vi "HFRR ADV v044.vi"() -> ()   [LabVIEW 2025] (continued)
            "LVDT MIN" <- w2060
            "LVDT MAX" <- w2059
            "LVDT Peak" <- w2058
            "pizo raw" <- w2057
            "cof" <- w2055
            "Frictioin Force Raw" <- w2056
          }
        }
      }
      frame Error {
      }
    }
    n1795 = local read "Quit"() -> (w1974:bool)
  }
  n1796 = disable-structure shown="Disabled" {
    disable-tunnel: errorcluster {"status"=TRUE, "code"=0, "source"="Init"} ("error IO") -> [w2119 _]
    disable-tunnel: [w2117 _] -> w50
    frame Disabled {
      n1797 = while {
        shift-right: [w2135] -> w2121
        shift-left: _ -> [w2126]
        shift-right: [w2134] -> w2120
        shift-left: w2119 -> [w2128]
        tunnel: [w2123] -> w2117
        tunnel: [w2133] -> _
        i -> [w2133]
        stop <- w2123 stop-if-true
        n1798 = local read "Port 1a"() -> (w2129:bool)
        n1799 = local read "Port 3"() -> (w2130:bool)
        n1800 = local read "Com Port 1"() -> (w2127:refnum<visa-resource-name>)
        n1801 = Or(x=w2130, y=w2129) -> (x .or. y?=w2132:bool)
        n1802 = Unbundle(w2128) -> ("status"=→"Port 3":bool)  [unwired: 2 out]
        n1803 = Not Equal?(x=w2127, y=w2126) -> (x != y?=w2124:bool)
        n1804 = case shown="True" w2132 {
          frame False {
            w2138 = TRUE ("Visible")
            n1805 = property on="Port 1a" class="Bool (strict)"("Visible"=w2138) -> ()  [unwired: 2 in, 2 out]
            n1806 = property on="Port 3" class="Bool (strict)"("Visible"=w2138) -> ()  [unwired: 2 in, 2 out]
          }
          frame True {
            w2139 = TRUE ("Visible")
            n1807 = property on="Port 1a" class="Bool (strict)"("Visible"=w2139) -> ()  [unwired: 2 in, 2 out]
            n1808 = property on="Port 3" class="Bool (strict)"("Visible"=w2139) -> ()  [unwired: 2 in, 2 out]
          }
        }
        n1809 = Wait (ms)(milliseconds to wait=u32 40) -> ()  [unwired: 1 out]
        n1810 = case shown="True" w2124 {
          tunnel: [w2136 errorcluster {"status"=TRUE, "code"=0, "source"="Init"} ("error out")] -> w2125
          tunnel: w2128 -> [w2136 _]
          frame False {
          }
          frame True {
          }
        }
        n1811 = case shown="Error" w2125 {
          selector: w2125 -> [w2146 w2164]
          tunnel: [w2149 w2168] -> w2135
          tunnel: [w2148 w2162] -> w2134
          tunnel: w2126 -> [w2147 w2166]
          frame No Error {
            n1812 = property class="Instr"(reference=w2147, error in=w2146) -> (reference out=w2144:refnum<visa-resource-name>, error out=w2145:errorcluster, "Serial Settings:Number of Bytes at Serial Port"=w2141:u32)
            n1813 = Greater?(x=w2141, y=u32 5) -> (0:w2140:bool)
            n1814 = Not(x=w2140) -> (.not. x?=→"Port 1a":bool)
            n1815 = while {
              tunnel: [w2157] -> w2148
              tunnel: [w2156] -> w2149
              tunnel: w2145 -> [w2155]
              tunnel: w2144 -> [w2154]
              stop <- TRUE stop-if-true
              n1816 = property class="Instr" props=["Serial Settings:Number of Bytes at Serial Port"](reference=w2154, error in=w2155) -> (reference out=w2159:refnum<visa-resource-name>, error out=w2158:errorcluster)  [unwired: 1 out]
              n1817 = VISA Read(VISA resource name=w2159, byte count=u32 50, error in (no error)=w2158) -> (VISA resource name out=w2156:refnum<visa-resource-name>, read buffer=w2151:string, error out=w2157:errorcluster)  [unwired: 1 out]
              n1818 = Wait (ms)(milliseconds to wait=u32 5) -> ()  [unwired: 1 out]
            }
          }
          frame Error {
            w2174 = u16 0 items=["None", "XON/XOFF", "RTS/CTS", "XON/XOFF & RTS/CTS", "DTR/DSR", "XON/XOFF & DTR/DSR"] ("flow control (0:none)  2")
            w2172 = u16 10 items=["1.0"=10, "1.5"=15, "2.0"=20] ("stop bits 2")
            w2170 = u16 0 items=["None", "Odd", "Even", "Mark", "Space"] ("parity 2")
            w2171 = u32 10000  # timeout (10sec)
            n1819 = VISA Close(VISA resource name=w2166, error in (no error)=w2164) -> (error out=w2167:errorcluster)
            n1820 = local write "Port 1a"(FALSE ("Port 1a")) -> ()
            n1821 = local read "Com Port 1"() -> (w2161:refnum<visa-resource-name>)
            n1822 = call <vilib>:"Clear Errors.vi"("error in (no error)"=w2167) -> ("error out"=w2165:errorcluster)  [unwired: 5 in, 1 out]
            n1823 = call-poly "VISA Configure Serial Port"("VISA resource name"=w2161, "timeout (10sec)"=w2171, "baud rate (9600)"=u32 250000 ("baud rate  2"), "data bits (8)"=u16 8 ("data bits  2"), "parity (0:none)"=w2170, "error in (no error)"=w2165, "stop bits (10: 1 bit)"=w2172, "flow control (0:none)"=w2174) -> ("VISA resource name out"=w2175:refnum<visa-resource-name>, "error out"=w2176:errorcluster)  [unwired: 6 in]
            n1824 = flat-sequence {
              tunnel: w2175 -> [w2178]
              tunnel: w2176 -> [w2177]
              tunnel: [w2178] -> w2168
              tunnel: [w2177] -> w2162
              frame #0 {
                n1825 = Wait (ms)(milliseconds to wait=u32 50) -> ()  [unwired: 1 out]
              }
            }
            "Residual Uno" <- ""
          }
        }
        n1826 = local read "Quit"() -> (w2123:bool)
        "Error Uno" <- w2128
      }
      n1827 = VISA Close(VISA resource name=w2121, error in (no error)=w2120) -> (error out=w2118:errorcluster)
      n1828 = call <vilib>:"Clear Errors.vi"("error in (no error)"=w2118) -> ()  [unwired: 5 in, 2 out]
    }
    frame Enabled {
    }
  }
  n1829 = while {
    stop <- w2189 stop-if-true
    # "V0OLTAGE TO STROKE (peice vise calibration)"
    n1830 = local read "LVDT MIN"() -> (w2181:dbl)
    n1831 = local read "LVDT Peak"() -> (w2180:dbl)
    n1832 = Wait (ms)(milliseconds to wait=u32 10) -> ()  [unwired: 1 out]
    n1833 = formula code="// Dynamic Parameterized Linear Interpolation Node\n// Inputs: vpp_val, voltages (Array), distances (Array)\n// Outputs: stroke\n\nint i = 0;\nint segments = 11; // 12 points make 11 interpolation segments\n\n// 1. Lower Boundary Clamp\nif (vpp_val <= voltages[0]) {\n    stroke = distances[0];\n}\n// 2. Upper Boundary Clamp\nelse if (vpp_val >= voltages[segments]) {\n    stroke = distances[segments];\n}\n// 3. Dynamic Segment Search Loop\nelse {\n    stroke = distances[0]; // Fallback baseline\n    for (i = 0; i < segments; i++) {\n        if (vpp_val >= voltages[i] && vpp_val <= voltages[i+1]) {\n            // Standard linear interpolation formula using array lookups\n            stroke = distances[i] + (vpp_val - voltages[i]) * (distances[i+1] - distances[i]) / (voltages[i+1] - voltages[i]);\n            break; // Segment found, safely exit the loop\n        }\n    }\n}"("vpp_val"=w2180, "voltages"="calibration values", "distances"="STROKE") -> ("stroke"=→"LVDT STROKE":dbl)
    n1834 = local read "Calibration Tare Value"() -> (w2185:dbl)
    n1835 = local read "Calibration Tare"() -> (w2183:bool)
    n1836 = Subtract(x=w2181, y=w2185) -> (x-y=→"LVDT STROKE  Calibration":dbl)
    n1837 = case shown="True" w2183 {
      selector: w2183 -> [_ w2191]
      tunnel: w2181 -> [_ w2192]
      frame False {
      }
      frame True {
        n1838 = Not(x=w2191) -> (.not. x?=w2190:bool)
        n1839 = local write "Calibration Tare"(w2190) -> ()
        "Calibration Tare Value" <- w2192
      }
    }
    n1840 = local read "Quit"() -> (w2189:bool)
  }
  n1841 = while {
    stop <- w2215 stop-if-true
    n1842 = local read "Due read"() -> (w2213:string)
    n1843 = call <vilib>:"High Resolution Polling Wait.vi"("seconds to wait"=0.02) -> ()  [unwired: 10 in, 1 out]
    n1844 = local read "Frictioin Force Raw"() -> (w2195:dbl)
    n1845 = Spreadsheet String To Array(delimiter (Tab)=";", format string="", spreadsheet string=w2213, array type (2D Dbl)=string[] []) -> (array=w2210:string[])
    n1846 = Fract/Exp String To Number(string=w2210) -> (number=w2209:dbl[])  [unwired: 3 in, 1 out]
    n1847 = call <vilib>:"Median Filter PtByPt.vi"("rank"=2, "x"=w2195) -> ("Filtered x"=→"Friction":dbl)  [unwired: 2 in, 1 out]
    n1848 = Index Array(array=w2209) -> (element #1=→"Sample Temperature 2":dbl, element #2=→"Target Sample Temperature":dbl, element #3=→"Current Duty Cycle":dbl, element #4=→"Ambient Temperature":dbl, element #5=→"Dac Status":dbl, element #6=→"Vpp":dbl, element #7=→"Active Error Code":dbl, element #8=→"Kp":dbl, element #9=→"Ki":dbl, element #10=→"Kd":dbl, element #11=→"SampleRaw":dbl, element #12=→"AmbRaw":dbl)  [unwired: 12 in]
    n1849 = local read "Quit"() -> (w2215:bool)
  }
  n1850 = while {
    shift-right: [w2229] -> w46
    shift-left: _ -> [w2221]
    shift-right: [w2216] -> w45
    shift-left: errorcluster {"status"=FALSE, "code"=0, "source"="Init"} ("error out") -> [w2223]
    tunnel: [w2218] -> w49
    tunnel: [w2228] -> _
    i -> [w2228]
    stop <- w2218 stop-if-true
    n1851 = local read "Com Port 2"() -> (w2222:refnum<visa-resource-name>)
    n1852 = local read "Port 2a"() -> (w2224:bool)
    n1853 = Unbundle(w2223) -> ("status"=→"Port 4":bool)  [unwired: 2 out]
    n1854 = call <vilib>:"High Resolution Polling Wait.vi"("seconds to wait"=0.02) -> ()  [unwired: 10 in, 1 out]
    n1855 = local read "Port 4"() -> (w2225:bool)
    n1856 = Not Equal?(x=w2222, y=w2221) -> (x != y?=w2220:bool)
    n1857 = Or(x=w2225, y=w2224) -> (x .or. y?=w2227:bool)
    n1858 = case shown="False" w2227 {
      frame False {
        w2232 = TRUE ("Visible")
        n1859 = property on="Port 2a" class="Bool (strict)"("Visible"=w2232) -> ()  [unwired: 2 in, 2 out]
        n1860 = property on="Port 4" class="Bool (strict)"("Visible"=w2232) -> ()  [unwired: 2 in, 2 out]
      }
      frame True {
        w2233 = TRUE ("Visible")
        n1861 = property on="Port 2a" class="Bool (strict)"("Visible"=w2233) -> ()  [unwired: 2 in, 2 out]
        n1862 = property on="Port 4" class="Bool (strict)"("Visible"=w2233) -> ()  [unwired: 2 in, 2 out]
      }
    }
    n1863 = case shown="True" w2220 {
      tunnel: [w2230 errorcluster {"status"=TRUE, "code"=0, "source"="Init"} ("error out")] -> w2219
      tunnel: w2223 -> [w2230 _]
      frame False {
      }
      frame True {
      }
    }
    n1864 = case shown="No Error" w2219 {
      selector: w2219 -> [w2246 w2277]
      tunnel: [w2239 w2282] -> w2229
      tunnel: [w2247 w2275] -> w2216
      tunnel: w2221 -> [w2248 w2280]
      frame No Error {
        n1865 = property class="Instr" props=["Serial Settings:Number of Bytes at Serial Port"](reference=w2248, error in=w2246) -> (reference out=w2240:refnum<visa-resource-name>, error out=w2245:errorcluster)  [unwired: 1 out]
        n1866 = while {
          tunnel: [w2256] -> w2241
          tunnel: [w2255] -> w2242
          tunnel: w2245 -> [w2254]
          tunnel: w2240 -> [w2253]
          tunnel: [w2252] -> _
          i -> [w2252]
          stop <- TRUE stop-if-true
          n1867 = property class="Instr" props=["Serial Settings:Number of Bytes at Serial Port"](reference=w2253, error in=w2254) -> (reference out=w2258:refnum<visa-resource-name>, error out=w2257:errorcluster)  [unwired: 1 out]
          n1868 = VISA Read(VISA resource name=w2258, byte count=u32 1000, error in (no error)=w2257) -> (VISA resource name out=w2255:refnum<visa-resource-name>, read buffer=→"Due read":string, error out=w2256:errorcluster)  [unwired: 1 out]
        }
        n1869 = local read "Due Write"() -> (w2238:string)
        n1870 = call <vilib>:"Trim Whitespace.vi"("string"=w2238) -> ("trimmed string"=w2237:string)  [unwired: 1 in]
        n1871 = Not Equal?(x=w2237, y="") -> (x != y?=w2243:bool)
        n1872 = VISA Flush I/O Buffer(VISA resource name=w2242) -> (VISA resource name out=w2235:refnum<visa-resource-name>, error out=→"error out 10":errorcluster)  [unwired: 2 in]
        n1873 = case shown="True" w2243 {
          tunnel: w2235 -> [w2260 w2265]
          tunnel: [w2260 w2269] -> w2239
          tunnel: w2241 -> [w2259 w2264]
          tunnel: [w2259 w2267] -> w2247
          tunnel: w2237 -> [_ w2263]
          tunnel: [_ w2266] -> _
          frame False {
            # "DATA  WRITE LOOP"
          }
          frame True {
            n1874 = Concatenate Strings(w2263, "\r\n") -> (w2262:string)
            n1875 = VISA Write(VISA resource name=w2265, write buffer=w2262, error in (no error)=w2264) -> (VISA resource name out=w2269:refnum<visa-resource-name>, return count=w2266:u32, error out=w2268:errorcluster)
            n1876 = flat-sequence {
              tunnel: w2268 -> [w2271]
              tunnel: [w2271] -> w2267
              frame #0 {
                n1877 = local write "Due Write"("" ("Command")) -> ()
                n1878 = Wait (ms)(milliseconds to wait=u32 5) -> ()  [unwired: 1 out]
              }
            }
          }
        }
        "Port 2a" <- TRUE ("Port 2a")
      }
      frame Error {
        w2288 = u16 0 items=["None", "XON/XOFF", "RTS/CTS", "XON/XOFF & RTS/CTS", "DTR/DSR", "XON/XOFF & DTR/DSR"] ("flow control (0:none)  2")
        w2286 = u16 10 items=["1.0"=10, "1.5"=15, "2.0"=20] ("stop bits 2")
        w2284 = u16 0 items=["None", "Odd", "Even", "Mark", "Space"] ("parity 2")
        w2285 = u32 10000  # timeout (10sec)
        n1879 = VISA Clear(VISA resource name=w2280, error in (no error)=w2277) -> (VISA resource name out=w2279:refnum<visa-resource-name>, error out=w2278:errorcluster)
        n1880 = VISA Close(VISA resource name=w2279, error in (no error)=w2278) -> (error out=w2281:errorcluster)
        n1881 = call <vilib>:"Clear Errors.vi"("error in (no error)"=w2281) -> ()  [unwired: 5 in, 2 out]
        n1882 = local write "Port 2a"(FALSE ("Port 2a")) -> ()
        n1883 = local read "Com Port 2"() -> (w2274:refnum<visa-resource-name>)
        "visa due" <- w2274
        n1884 = call-poly "VISA Configure Serial Port"("VISA resource name"=w2274, "timeout (10sec)"=w2285, "baud rate (9600)"=u32 250000 ("baud rate  2"), "data bits (8)"=u16 8 ("data bits  2"), "parity (0:none)"=w2284, "stop bits (10: 1 bit)"=w2286, "flow control (0:none)"=w2288) -> ("VISA resource name out"=w2289:refnum<visa-resource-name>, "error out"=w2290:errorcluster)  [unwired: 7 in]
        n1885 = flat-sequence {
          tunnel: w2289 -> [w2292]
          tunnel: w2290 -> [w2291]
          tunnel: [w2292] -> w2282
          tunnel: [w2291] -> w2275
          frame #0 {
            n1886 = Wait (ms)(milliseconds to wait=u32 50) -> ()  [unwired: 1 out]
          }
        }
        "Residual Due" <- ""
      }
    }
    "error out 9" <- w2216
    n1887 = local read "Quit"() -> (w2218:bool)
    "Error Due" <- w2223
  }
  n1888 = local write "FRICVALZ"(0.0 ("FRICVALZ")) -> ()
  n1889 = property on="RUN" class="Bool (strict)"("Visible"=TRUE) -> ()  [unwired: 2 in, 2 out]
  n1890 = while {
    tunnel: [w2307] -> _
    tunnel: [w2294] -> w59
    i -> [w2307]
    stop <- w2294 stop-if-true
    n1891 = local read "conststatus"() -> (w2298:dbl)
    n1892 = local read "Main Tab"() -> (w2296:T4)
    n1893 = local read "EDIT"() -> (w2313:bool)
    n1894 = local read "Rate"() -> (w2312:dbl)
    n1895 = case shown="True" w2313 {
      tunnel: [FALSE TRUE] -> _
      frame False {
      }
      frame True {
      }
    }
    n1896 = Equal?(x=w2296, y=T28."About" ("Main Tab")) -> (x = y?=w2305:bool)
    n1897 = Equal?(x=w2298, y=0.0) -> (x = y?=w2299:bool)
    n1898 = Divide(x=1.0, y=w2312) -> (x/y=w2308:dbl)
    "Time 2" <- w2308
    n1899 = case shown="True" w2299 {
      frame False {
      }
      frame True {
        # "C:\\WinDucom\\calibrate WO 2391.dcf"
        n1900 = local write "Lan flag"(22) -> ()
        n1901 = local write "conststatus"(10.0 ("rpm value : 2")) -> ()
        n1902 = String To Path(string="C:\\LAB-IQ\\calibrate WO 2465.dcf") -> (path=w2319:path)
        n1903 = Open/Create/Replace File "Open File"(file path (use dialog)=w2319) -> (refnum out=w2317:refnum<file>)  [unwired: 5 in, 2 out]
        n1904 = for {
          N: 23 -> [_]
          tunnel: w2317 -> [w2328]
          i -> [w2322]
          (unwired) TRUE ("line mode (F)")
          n1905 = Read from Text File "Read File"(file (use dialog)=w2328) -> (text=w2327:string)  [unwired: 3 in, 3 out]
          n1906 = Match Pattern(string=w2327, regular expression="]") -> (after substring=w2325:string)  [unwired: 1 in, 3 out]
          n1907 = String Subset(string=w2327, offset (0)=5, length (rest)=10 ("length (rest)")) -> (substring=w2320:string)
          n1908 = Fract/Exp String To Number(string=w2320) -> (number=w2321:dbl)  [unwired: 3 in, 1 out]
          n1909 = Match Pattern(string=w2325, regular expression="-") -> (before substring=w2323:string)  [unwired: 1 in, 3 out]
          n1910 = case shown="10" w2322 {
            tunnel: w2321 -> [_ _ _ _ _ _ _ _ _ _ w2335 _ _ _ _ _ _ _ _ _ _ _ _ _]
            tunnel: w2323 -> [_ _ _ _ w2331 w2332 w2333 _ _ _ _ _ _ _ _ _ _ _ _ _ w2336 w2337 w2338 _]
            frame 0 {
            }
            frame 1 {
            }
            frame 2 {
            }
            frame 3 {
            }
            frame 4 {
              n1911 = local write "Com Port 1"(w2331) -> ()
            }
            frame 5 {
              n1912 = local write "Com Port 2"(w2332) -> ()
              n1913 = local write "visa due"(w2332) -> ()
            }
            frame 6 {
              n1914 = String To Path(string=w2333) -> (path=w2334:path)
              n1915 = local write "File Path"(w2334) -> ()
              "String" <- w2333
            }
            frame 7 {
            }
            frame 8 {
            }
            frame 9 {
            }
            frame 10 {
              n1916 = local write "Language Selection"(w2335) -> ()
            }
            frame 11 {
            }
            frame 12 {
            }
            frame 13 {
            }
            frame 14 {
            }
            frame 15 {
            }
            frame 16 {
            }
            frame 17 {
            }
            frame 18 {
            }
            frame 21 {
            }
            frame 22 {
              n1917 = local write "Com Port 3"(w2336) -> ()
            }
            frame 20 {
              n1918 = local write "Camera Port :"(w2337) -> ()
            }
            frame 19 {
              n1919 = local write "C3 :"(w2338) -> ()
            }
            frame 23, Default {
            }
          }
        }
      }
    }
    n1920 = Select(t=u32 2500 ("milliseconds to wait"), s=w2305, f=u32 500 ("milliseconds to wait")) -> (s? t:f=w2303:u32)
    n1921 = Multiply(x=w2308, y=w2303) -> (x*y=w2310:dbl)
    n1922 = call "Elapsed Time2"("Time Target (s)"=w2310, "Auto Reset"=TRUE) -> ("Time has Elapsed"=w2300:bool)  [unwired: 10 in, 7 out]
    n1923 = case shown="True" w2300 {
      frame False {
      }
      frame True {
        n1924 = stacked-sequence {
          frame #0 {
            # "DATA PROCESSING"
            # "115 mV/N"
            n1925 = local read "Sample Temperature 2"() -> (w2341:dbl)
            n1926 = local read "RH Numeric:"() -> (→"Humidity ( %RH )":dbl)
            n1927 = local read "FRICVALZ"() -> (w2358:dbl)
            n1928 = local read "Friction"() -> (w2344:dbl)
            n1929 = call <vilib>:"Mean PtByPt.vi"("x"=w2341, "sample length"=100) -> ("mean"=w2340:dbl)  [unwired: 2 in, 1 out]
            "TEMP 2" <- w2340
            "TEMP 3" <- w2340
            n1930 = Subtract(x=w2344, y=w2358) -> (x-y=w2353:dbl)
            "FF 2" <- w2353
            "FF 4" <- w2353
            n1931 = local read "Ambient Temperature"() -> (→"AIR TEMP":dbl)
            n1932 = local read "TEMP"() -> (w2357:dbl)
            n1933 = local write "FF 3"(w2353) -> ()
            n1934 = Compound Arithmetic op=OR("FRICVALZ 4", "FRICVALZ 3", "FRICVALZ 2") -> (w2349:bool)
            n1935 = case shown="True" w2349 {
              tunnel: w2344 -> [_ w2364]
              frame False {
              }
              frame True {
                w2363 = FALSE ("FRICVALZ")
                n1936 = local write "FRICVALZ 3"(w2363) -> ()
                n1937 = local write "FRICVALZ 2"(w2363) -> ()
                n1938 = local write "FRICVALZ 4"(w2363) -> ()
                "FRICVALZ" <- w2364
              }
            }
            n1939 = Not A Number/Path/Refnum?(number/path/refnum=w2357) -> (NaN/Path/Refnum?=w2356:bool)
            n1940 = Not A Number/Path/Refnum?(number/path/refnum=w2353) -> (NaN/Path/Refnum?=w2355:bool)
            n1941 = Divide(x=w2353, y=1.96) -> (x/y=w2350:dbl)
            n1942 = Compound Arithmetic op=OR(w2356, w2355) -> (w2354:bool)
            n1943 = Not A Number/Path/Refnum?(number/path/refnum=w2350) -> (NaN/Path/Refnum?=w2351:bool)
            n1944 = case shown="True" w2354 {
              frame False {
              }
              frame True {
                n1945 = local write "TEMP"(0.0 ("TEMP")) -> ()
                n1946 = local write "FF 2"(0.0 ("FF 2")) -> ()
                n1947 = local write "reinit"(TRUE ("reinit")) -> ()
              }
            }
            n1948 = local write "TEMP"(w2340) -> ()
            n1949 = Select(t=0.0, s=w2351, f=w2350) -> (s? t:f=w2343:dbl)
            "COF 2" <- w2343
            n1950 = local write "COF 3"(w2343) -> ()
          }
        }
      }
    }
    n1951 = Wait (ms)(milliseconds to wait=u32 50) -> ()  [unwired: 1 out]
    n1952 = local read "Quit"() -> (w2294:bool)
    "Rate" <- 2500.0 ("No of Samples")
  }
  n1953 = while {
    tunnel: [w2384] -> _
    tunnel: [w2367] -> w61
    tunnel: w6 -> [_]
    i -> [w2384]
    stop <- w2367 stop-if-true
    # "C:\\LAB-IQ-NXT\\Scar View.exe"
    n1954 = local read "OK Button 16"() -> (w2374:bool)
    n1955 = local read "Main Tab"() -> (w2368:T4)
    n1956 = local read "service 3"() -> (w2369:bool)
    n1957 = local read "OPEN 6"() -> (w2371:bool)
    n1958 = local read "EDIT 2"() -> (w2373:bool)
    n1959 = flat-sequence {
      frame #0 {
        n1960 = stacked-sequence {
          frame #0 {
            n1961 = local read "EDIT"() -> (w2862:bool)
            n1962 = case shown="False" w2862 {
              tunnel: [u8 2 ("Disabled") u8 0 ("Disabled")] -> _
              frame False {
                w2864 = FALSE
                n1963 = local write "Password"("") -> ()
                n1964 = local write "x = y?"(w2864) -> ()
                n1965 = property on="Password" class="Str"("Visible"=w2864) -> ()  [unwired: 2 in, 2 out]
              }
              frame True {
                n1966 = property on="Password" class="Str"("Visible"=TRUE) -> ()  [unwired: 2 in, 2 out]
              }
            }
            "dipl pwd" <- "@143$\n" ("dipl pwd")
          }
          frame #1 {
          }
          frame #2 {
          }
          frame #3 {
          }
          frame #4 {
            n1967 = String To Byte Array(string="Password") -> (unsigned byte array=w2875:u8[])
            n1968 = Search 1D Array(1D array=w2875, element=u8 10) -> (index of element=w2873:i32)  [unwired: 1 in]
            n1969 = Index Array(array=w2875, index=w2873) -> (element=w2874:u8)
            n1970 = Equal?(x=w2874, y=10) -> (x = y?=w2870:bool)
            n1971 = case shown="True" w2870 {
              frame False {
              }
              frame True {
                # "password"
                # "password"
                n1972 = local read "Password"() -> (w2887:string)
                n1973 = String To Byte Array(string=w2887) -> (unsigned byte array=w2890:u8[])
                n1974 = String To Byte Array(string="@143$\n") -> (unsigned byte array=w2877:u8[])
                n1975 = Array Size(array=w2890) -> (size(s)=w2886:i32)
                n1976 = Array Size(array=w2877) -> (size(s)=w2882:i32)
                n1977 = for {
                  N: w2886 -> [_]
                  tunnel: w2890 -> [w2903]
                  tunnel: [w2901] -> w2891 mode=indexing
                  tunnel: w2886 -> [w2898]
                  i -> [w2899]
                  n1978 = Decrement(x=w2898) -> (x-1=w2897:i32)
                  n1979 = Index Array(array=w2903, index=w2899) -> (element=w2902:u8)
                  n1980 = Equal?(x=w2899, y=w2897) -> (x = y?=w2896:bool)
                  n1981 = Number To Decimal String(number=w2902) -> (decimal integer string=w2900:string)  [unwired: 1 in]
                  n1982 = Select(t="", s=w2896, f="\r") -> (s? t:f=w2893:string)
                  n1983 = Concatenate Strings(w2900, w2893) -> (w2901:string)
                }
                n1984 = for {
                  N: w2882 -> [_]
                  tunnel: w2877 -> [w2914]
                  tunnel: [w2912] -> w2880 mode=indexing
                  tunnel: w2882 -> [w2909]
                  i -> [w2910]
                  n1985 = Decrement(x=w2909) -> (x-1=w2908:i32)
                  n1986 = Index Array(array=w2914, index=w2910) -> (element=w2913:u8)
                  n1987 = Equal?(x=w2910, y=w2908) -> (x = y?=w2907:bool)
                  n1988 = Number To Decimal String(number=w2913) -> (decimal integer string=w2911:string)  [unwired: 1 in]
                  n1989 = Select(t="", s=w2907, f="\r") -> (s? t:f=w2904:string)
                  n1990 = Concatenate Strings(w2911, w2904) -> (w2912:string)
                }
                n1991 = local read "file path"() -> (w2876:path)
                n1992 = call <vilib>:"Read Characters From File.vi"("file path (dialog if empty)"=w2876) -> ("character string"=w2889:string)  [unwired: 5 in, 3 out]
                "string" <- w2889
                n1993 = flat-sequence {
                  tunnel: [w2892] -> _
                  frame #0 {
                    w2892 = ""
                    n1994 = local write "Password"(w2892) -> ()
                  }
                }
                n1995 = Concatenate Strings(w2880) -> (w2881:string)
                n1996 = Concatenate Strings(w2889) -> (w2888:string)
                n1997 = Concatenate Strings(w2891) -> (w2884:string)
                n1998 = Equal?(x=w2884, y=w2888) -> (x = y?=w2879:bool)
                n1999 = Equal?(x=w2884, y=w2881) -> (x = y?=w2885:bool)
                n2000 = Or(x=w2879, y=w2885) -> (x .or. y?=→"x = y?":bool)
              }
            }
          }
        }
        n2001 = local read "x = y?"() -> (w2860:bool)
        n2002 = And(x="EDIT", y=w2860) -> (x .and. y?=w2858:bool)
        n2003 = case shown="True" w2858 {
          tunnel: [u8 2 ("Disabled") u8 0 ("Disabled")] -> w2857
          tunnel: [w3064 TRUE ("Visible")] -> w2856
          frame False {
            w3064 = FALSE ("Visible")
            n2004 = local write "EDIT 2"(w3064) -> ()
          }
          frame True {
          }
        }
        n2005 = case shown="True" "SAVE" {
          frame False {
          }
          frame True {
            n2006 = stacked-sequence {
              seq-local: [w2919 _ _] -> [_ w3060 _]
              frame #0 {
                w2915 = 0.0 ("number")
                w2916 = 0.0 ("number")
                (unwired) i16 5 ("precision (6)")
                # "[CH1]    - FF\n[CH2]   - TEMPERATURE\n[CH3]    - Humidity\n[CH4]    - AIR TEMP\n[CH5]\\- Visa Uno\n[CH6] \\- Visa Due\n[CH7]  \\- file path\n[CH8]   - Displacement Gain\n[CHA]   - Stroke Gain\n[CHB]   - Stroke PID Gain\n[CHC]   -Language Selection\n[CHD]   -Power +\n[CHE]   -Power_\n[CHF]   -Heater\n[CHG]   -Humidity Wet\n[CHH]   -Humidity Dry\n[CHI]   -Integral Time"
                n2007 = local read "Language Selection"() -> (w2962:enum16{"English", "Russian"})
                n2008 = Path To String(path="File Path") -> (string=w2978:string)
                n2009 = Number To Fractional String(number=w2915, width (-)=i16 10 ("precision (6)"), precision (6)=i16 5) -> (F-format string=w2969:string)  [unwired: 1 in]
                n2010 = Number To Fractional String(number=w2962, width (-)=i16 10 ("precision (6)"), precision (6)=i16 5) -> (F-format string=w2958:string)  [unwired: 1 in]
                n2011 = Number To Fractional String(number=w2916, width (-)=i16 10 ("precision (6)"), precision (6)=i16 5) -> (F-format string=w2952:string)  [unwired: 1 in]
                n2012 = Number To Fractional String(number=w2916, width (-)=i16 10 ("precision (6)"), precision (6)=i16 5) -> (F-format string=w2949:string)  [unwired: 1 in]
                n2013 = Number To Fractional String(number=w2916, width (-)=i16 10 ("precision (6)"), precision (6)=i16 5) -> (F-format string=w2944:string)  [unwired: 1 in]
                n2014 = Number To Fractional String(number=w2916, width (-)=i16 10 ("precision (6)"), precision (6)=i16 5) -> (F-format string=w2941:string)  [unwired: 1 in]
                n2015 = Number To Fractional String(number=w2916, width (-)=i16 10 ("precision (6)"), precision (6)=i16 5) -> (F-format string=w2936:string)  [unwired: 1 in]
                n2016 = local read "Com Port 1"() -> (w2918:refnum<visa-resource-name>)
                n2017 = local read "Com Port 2"() -> (w2917:refnum<visa-resource-name>)
                n2018 = Concatenate Strings(w2978, "\\" ("string")) -> (w2977:string)
                n2019 = Number To Fractional String(number=w2915, width (-)=i16 10 ("precision (6)"), precision (6)=i16 5) -> (F-format string=w3010:string)  [unwired: 1 in]
                n2020 = Number To Fractional String(number=w2915, width (-)=i16 10 ("precision (6)"), precision (6)=i16 5) -> (F-format string=w3009:string)  [unwired: 1 in]
                n2021 = Number To Fractional String(number=w2915, width (-)=i16 10 ("precision (6)"), precision (6)=i16 5) -> (F-format string=w3003:string)  [unwired: 1 in]
                n2022 = Number To Fractional String(number=w2915, width (-)=i16 10 ("precision (6)"), precision (6)=i16 5) -> (F-format string=w2997:string)  [unwired: 1 in]
                n2023 = Number To Fractional String(number=w2915, width (-)=i16 10 ("precision (6)"), precision (6)=i16 5) -> (F-format string=w2970:string)  [unwired: 1 in]
                n2024 = Concatenate Strings("[CHA]" ("string"), w2969, "- Stroke Gain" ("string"), "\r") -> (w2963:string)
                n2025 = Concatenate Strings("[CHC]" ("string"), w2958, "-Language Selection" ("string"), "\r") -> (w2955:string)
                n2026 = Concatenate Strings("[CHD]" ("string"), w2952, "-Power +" ("string"), "\r") -> (w2934:string)
                n2027 = Concatenate Strings("[CHG]" ("string"), w2941, "-Humidity Wet" ("string"), "\r") -> (w2931:string)
                n2028 = Concatenate Strings("[CHH]" ("string"), w2936, "-Humidity Dry" ("string"), "\r") -> (w2930:string)
                n2029 = Concatenate Strings("[CH1]" ("string"), w3010, " - FF" ("string"), "\r") -> (w3008:string)
                n2030 = Concatenate Strings("[CH2]" ("string"), w3009, " - TEMPERATURE" ("string"), "\r") -> (w3007:string)
                n2031 = Concatenate Strings("[CH3]" ("string"), w3003, " - Humidity" ("string"), "\r") -> (w3000:string)
                n2032 = Concatenate Strings("[CH4]" ("string"), w2997, " - AIR TEMP" ("string"), "\r") -> (w2993:string)
                n2033 = Concatenate Strings("[CH5]" ("string"), w2918, "- Visa Uno" ("string"), "\r") -> (w2986:string)
                n2034 = Concatenate Strings("[CH6]" ("string"), w2917, "- Visa Due" ("string"), "\r") -> (w2981:string)
                n2035 = Concatenate Strings("[CH7]" ("string"), w2977, "- file path" ("string"), "\r") -> (w2980:string)
                n2036 = Concatenate Strings("[CH8]" ("string"), w2970, "- Displacement Gain" ("string"), "\r") -> (w2973:string)
                n2037 = Concatenate Strings("[CHE]" ("string"), w2949, "-Power_" ("string"), "\r") -> (w2933:string)
                n2038 = Concatenate Strings("[CHF]" ("string"), w2944, "-Heater" ("string"), "\r") -> (w2932:string)
                n2039 = Concatenate Strings(w3008, w3007, w3000, w2993, w2986, w2981, w2980, w2973, w2963, w2955, w2934, w2933, w2932, w2931, w2930) -> (w2919:string)
                "gain" <- w2919
              }
              frame #1 {
                w3021 = 0.0 ("number")
                n2040 = local read "Camera Port :"() -> (w3024:string)
                n2041 = local read "C3 :"() -> (w3032:refnum<visa-resource-name>)
                n2042 = local read "Com Port 3"() -> (w3033:refnum<visa-resource-name>)
                n2043 = Concatenate Strings("[CH8]" ("string"), w3024, "- Visa Camera" ("string"), "\r") -> (w3023:string)
                n2044 = Concatenate Strings("[CH7]" ("string"), w3032, "- Visa Humidity" ("string"), "\r") -> (w3028:string)
                n2045 = Number To Fractional String(number=w3021, width (-)=i16 10 ("precision (6)"), precision (6)=i16 5) -> (F-format string=w3048:string)  [unwired: 1 in]
                n2046 = Concatenate Strings("[CHL]" ("string"), w3033, "- Visa humid" ("string"), "\r") -> (w3036:string)
                n2047 = Number To Fractional String(number=w3021, width (-)=i16 10 ("precision (6)"), precision (6)=i16 5) -> (F-format string=w3055:string)  [unwired: 1 in]
                n2048 = Concatenate Strings("[CHK]" ("string"), w3048, "-TEMP INTERCEPT" ("string"), "\r") -> (w3044:string)
                n2049 = Concatenate Strings("[SNO]" ("string"), "" ("string"), "-" ("string"), "\r") -> (w3041:string)
                n2050 = Concatenate Strings("[CHJ]" ("string"), w3055, "-AIR TEMP INTERCEPT" ("string"), "\r") -> (w3045:string)
                n2051 = String To Path(string="C:\\LAB-IQ\\calibrate WO 2465.dcf") -> (path=w3034:path)
                n2052 = Concatenate Strings(w3060, w3045, w3044, w3041, w3036, w3028, w3023) -> (w3059:string)
                n2053 = call <vilib>:"Write Characters To File.vi"("append to file? (new file:F)"=FALSE, "character string"=w3059, "file path (dialog if empty)"=w3034) -> ()  [unwired: 2 in, 1 out]
              }
              frame #2 {
                n2054 = local write "Lan flag"(0.0 ("Lan flag")) -> ()
                n2055 = local write "conststatus"(0.0 ("rpm value : 2")) -> ()
                n2056 = local write "SAVE"(FALSE ("OK Button 14")) -> ()
              }
            }
          }
        }
        n2057 = property on="EDIT 2" class="Bool (strict)"("Visible"=w2856) -> ()  [unwired: 2 in, 2 out]
        n2058 = property on="SAVE" class="Bool (strict)"("Visible"=w2856) -> ()  [unwired: 2 in, 2 out]
        n2059 = property on="visa due" class="CmbBox"("Disabled"=w2857) -> ()  [unwired: 2 in, 2 out]
        n2060 = property on="File Path" class="Path"("Disabled"=w2857) -> ()  [unwired: 2 in, 2 out]
        n2061 = property on="Language Selection" class="Enum (strict)"("Visible"=w2856) -> ()  [unwired: 2 in, 2 out]
        n2062 = property on="SPEED OUT:" class="DigNum (strict)"("Disabled"=w2857) -> ()  [unwired: 2 in, 2 out]
      }
    }
    n2063 = local read "RUN"() -> (w2383:bool)
    n2064 = local read "RUN"() -> (w2381:bool)
    n2065 = case shown="True" "EDIT 3" {
      frame False {
      }
      frame True {
        n2066 = local write "EDIT 3"(FALSE ("EDIT 3")) -> ()
        n2067 = local write "Main Tab"(T4."About" ("Main Tab")) -> ()
      }
    }
    n2068 = case shown="False" w2383 {
      frame False {
        n2069 = local read "stopT"() -> (w3071:bool)
        n2070 = case shown="True" w3071 {
          frame False {
          }
          frame True {
            n2071 = local write "stopT"(FALSE) -> ()
          }
        }
      }
      frame True {
        "stopT" <- TRUE
      }
    }
    n2072 = case shown="False" w2381 {
      frame False {
      }
      frame True {
      }
    }
    n2073 = case shown="True" w2373 {
      frame False {
        n2074 = property on="Password 2" class="Str"("Visible"=FALSE) -> ()  [unwired: 2 in, 2 out]
        n2075 = local write "Password 2"("" ("Password")) -> ()
      }
      frame True {
        n2076 = property on="Password 2" class="Str"("Visible"=TRUE) -> ()  [unwired: 2 in, 2 out]
        n2077 = Equal?(x="Password 2", y="HFRR1234") -> (x = y?=w2396:bool)
        n2078 = case shown="True" w2396 {
          tunnel: "Password 2" -> [w2399 _]
          frame False {
            n2079 = String Length(string=w2399) -> (length=w2400:i32)
            n2080 = Greater Than 0?(x=w2400) -> (x > 0?=w2398:bool)
            n2081 = case shown="False" w2398 {
              frame False {
                n2082 = property on="Password 2" class="Str"("Caption.Text"="Password (Advance Setting)") -> ()  [unwired: 2 in, 2 out]
              }
              frame True {
                n2083 = property on="Password 2" class="Str"("Caption.Text"="Incorrect Password!") -> ()  [unwired: 2 in, 2 out]
              }
            }
          }
          frame True {
            n2084 = local write "EDIT 2"(FALSE ("EDIT 2")) -> ()
            n2085 = local write "Password 2"("" ("Password")) -> ()
            n2086 = local write "Main Tab"(T4."Advance" ("Main Tab")) -> ()
            n2087 = local write "Main Dashboard Buttons"(T1."Advance" ("Main Dashboard Buttons")) -> ()
          }
        }
      }
    }
    n2088 = case shown="True" "Prog Uno" {
      frame False {
      }
      frame True {
        n2089 = stacked-sequence {
          frame #0 {
            n2090 = Delete(path (use dialog)=path "C:/LAB-IQ-NXT/UNOCOMPILE.bat" ("working directory")) -> ()  [unwired: 4 in, 3 out]
          }
          frame #1 {
            n2091 = local read "Com Port 1"() -> (w2838:refnum<visa-resource-name>)
            n2092 = Concatenate Strings("cmd.exe /c \"mode " ("command line"), w2838, ":1200,n,8,1\"\n" ("command line")) -> (w2843:string)
            n2093 = Concatenate Strings(w2843, "CD\\\nCD WinDucom\navrdude -C avrdude.conf -v -patmega328p -carduino -P" ("command line"), w2838, " -b115200 -D -Uflash:w:UNO_V20.hex:i\n" ("command line"), "\r") -> (w2845:string)
            "STR" <- w2845
            n2094 = call <vilib>:"Write Characters To File.vi"("append to file? (new file:F)"=FALSE, "character string"=w2845, "file path (dialog if empty)"=path "C:/LAB-IQ/UNOCOMPILE.bat" ("working directory")) -> ()  [unwired: 2 in, 1 out]
          }
          frame #2 {
            n2095 = disable-structure shown="Disabled" {
              frame Disabled {
                w2849 = "cmd.exe  /c \"C:\\LAB-IQ-NXT\\UNOCOMPILE.bat\"" ("string")
                n2096 = local write "Prog Uno"(FALSE ("run minimized? (F)")) -> ()
                n2097 = call <vilib>:"System Exec.vi"("expected output size  (4096)"=u32 65535, "run minimized? (F)"=FALSE, "wait until completion? (T)"=TRUE ("run minimized? (F)"), "working directory"=path "C:/LAB-IQ-NXT", "standard input"=w2849, "command line"=w2849) -> ("error out"=w2848:errorcluster, "standard output"=→"String 42":string)  [unwired: 2 in, 2 out]
                "error out 3" <- w2848
                n2098 = flat-sequence {
                  tunnel: w2848 -> [_]
                  frame #0 {
                  }
                }
              }
              frame Enabled {
              }
            }
          }
        }
      }
    }
    n2099 = case shown="\"ISO 12156\"" "TEST STANDARD" {
      frame "ASTM D6079", Default {
        w2818 = 50.0 ("Hz")
        w2819 = 53.0 ("Set Rh")
        w2821 = 1.0 ("Set Strk")
        w2820 = 60.0 ("Set Temp")
        # "astm hide"
        n2100 = local write "NORMAL LOAD"(200.0 ("NORMAL LOAD")) -> ()
        n2101 = local write "Set Strk"(w2821) -> ()
        n2102 = local write "Set Hz"(w2818) -> ()
        n2103 = local write "Set Temp"(w2820) -> ()
        n2104 = local write "Set Rh"(w2819) -> ()
        n2105 = local write "test time"(75.0 ("test time")) -> ()
        n2106 = local write "Set Stroke:"(w2821) -> ()
        n2107 = local write "Set Humidity:"(w2819) -> ()
        n2108 = local write "Set Frequency:"(w2818) -> ()
        n2109 = local write "Set Temperature:"(w2820) -> ()
        "Test Standard" <- "ASTM D6079" ("Test Standard 2")
      }
      frame "ISO 12156" {
        n2110 = local write "Set Strk"(1.0 ("Set Strk")) -> ()
        n2111 = local write "NORMAL LOAD"(200.0 ("NORMAL LOAD")) -> ()
        n2112 = local write "Set Temp"(60.0 ("Set Temp")) -> ()
        n2113 = local write "test time"(75.0 ("test time")) -> ()
        n2114 = local write "Set Hz"(50.0 ("Hz")) -> ()
        n2115 = local write "Set Rh"(53.0 ("Set Rh")) -> ()
      }
      frame "CEC F-096-A-06" {
        n2116 = local write "Set Strk"(1.0 ("Set Strk")) -> ()
        n2117 = local write "NORMAL LOAD"(200.0 ("NORMAL LOAD")) -> ()
        n2118 = local write "Set Temp"(60.0 ("Set Temp")) -> ()
        n2119 = local write "test time"(75.0 ("test time")) -> ()
        n2120 = local write "Set Hz"(50.0 ("Hz")) -> ()
        n2121 = local write "Set Rh"(53.0 ("Set Rh")) -> ()
      }
      frame "Custom" {
      }
    }
    n2122 = Or(x=w2371, y=w2369) -> (x .or. y?=w2370:bool)
    n2123 = case shown="\"About\"" w2368 {
      tunnel: [T28."Acquire" ("Main Tab") T28."Compare Files" ("Main Tab") T28."About" ("Main Tab")] -> w2379
      frame "Acquire", Default {
      }
      frame "Compare Files" {
      }
      frame "About" {
      }
    }
    n2124 = Or(x=w2374, y="OPEN") -> (x .or. y?=w2375:bool)
    n2125 = case shown="True" w2375 {
      tunnel: w2374 -> [_ w2407]
      frame False {
      }
      frame True {
        n2126 = stacked-sequence {
          tunnel: w2407 -> [_ w2474 _ _]
          frame #0 {
            w2423 = "  " ("String 6")
            n2127 = local write "OPEN"(FALSE ("open")) -> ()
            n2128 = local read "string1 2"() -> (w2411:string)
            n2129 = local read "string1 3"() -> (w2410:string)
            n2130 = local read "string1 4"() -> (w2409:string)
            n2131 = property on="OPEN" class="Bool (strict)"("Visible"=FALSE) -> ()  [unwired: 2 in, 2 out]
            n2132 = local write "String 6"(w2423) -> ()
            n2133 = local write "String 7"(w2423) -> ()
            n2134 = local write "String 8"(w2423) -> ()
            n2135 = local write "String 12"(w2423) -> ()
            n2136 = local read "OK Button 16"() -> (w2408:bool)
            n2137 = String To Path(string=w2411) -> (path=w2419:path)
            n2138 = String To Path(string=w2410) -> (path=w2418:path)
            n2139 = String To Path(string=w2409) -> (path=w2417:path)
            n2140 = case shown="True" w2408 {
              tunnel: [w2424 w2425] -> w2412
              frame False {
                n2141 = local read "string1"() -> (w2424:string)
              }
              frame True {
                n2142 = local read "String Indicator 4"() -> (w2425:string)
              }
            }
            n2143 = Open/Create/Replace File "Open File"(file path (use dialog)=w2419) -> (refnum out=w2415:refnum<file>)  [unwired: 5 in, 2 out]
            n2144 = Open/Create/Replace File "Open File"(file path (use dialog)=w2418) -> (refnum out=w2414:refnum<file>)  [unwired: 5 in, 2 out]
            n2145 = Open/Create/Replace File "Open File"(file path (use dialog)=w2417) -> (refnum out=w2413:refnum<file>)  [unwired: 5 in, 2 out]
            n2146 = while {
              tunnel: w2415 -> [w2437]
              i -> [w2433]
              stop <- w2432 continue-if-true
              (unwired) TRUE ("line mode (F)")
              n2147 = Read from Text File "Read File"(file (use dialog)=w2437) -> (text=w2434:string)  [unwired: 3 in, 3 out]
              n2148 = local write "Numeric 11"(w2433) -> ()
              n2149 = String Length(string=w2434) -> (length=w2436:i32)
              n2150 = Greater?(x=w2436, y=1) -> (0:w2432:bool)
            }
            n2151 = while {
              tunnel: w2414 -> [w2443]
              i -> [w2439]
              stop <- w2438 continue-if-true
              (unwired) TRUE ("line mode (F)")
              n2152 = Read from Text File "Read File"(file (use dialog)=w2443) -> (text=w2440:string)  [unwired: 3 in, 3 out]
              n2153 = local write "Numeric 12"(w2439) -> ()
              n2154 = String Length(string=w2440) -> (length=w2442:i32)
              n2155 = Greater?(x=w2442, y=1) -> (0:w2438:bool)
            }
            n2156 = while {
              tunnel: w2413 -> [w2449]
              i -> [w2445]
              stop <- w2444 continue-if-true
              (unwired) TRUE ("line mode (F)")
              n2157 = Read from Text File "Read File"(file (use dialog)=w2449) -> (text=w2446:string)  [unwired: 3 in, 3 out]
              n2158 = local write "Numeric 13"(w2445) -> ()
              n2159 = String Length(string=w2446) -> (length=w2448:i32)
              n2160 = Greater?(x=w2448, y=1) -> (0:w2444:bool)
            }
            n2161 = String To Path(string=w2412) -> (path=w2420:path)
            n2162 = Open/Create/Replace File "Open File"(file path (use dialog)=w2420) -> (refnum out=w2416:refnum<file>)  [unwired: 5 in, 2 out]
            n2163 = while {
              tunnel: w2416 -> [w2431]
              i -> [w2427]
              stop <- w2426 continue-if-true
              (unwired) TRUE ("line mode (F)")
              n2164 = Read from Text File "Read File"(file (use dialog)=w2431) -> (text=w2428:string)  [unwired: 3 in, 3 out]
              n2165 = local write "Numeric 8"(w2427) -> ()
              n2166 = String Length(string=w2428) -> (length=w2430:i32)
              n2167 = Greater?(x=w2430, y=1) -> (0:w2426:bool)
            }
          }
          frame #1 {
            w2601 = FALSE ("ACTUAL   MERGE")
            # "Sample Temp"
            # "ECR"
            # "COF"
            # "Time\nCOF\nFF\nTemp"
            n2168 = case shown="True" w2474 {
              tunnel: [w2621 w2622] -> w2475
              frame False {
                n2169 = local read "string1"() -> (w2621:string)
              }
              frame True {
                n2170 = local read "String Indicator 4"() -> (w2622:string)
              }
            }
            n2171 = local read "string1 3"() -> (w2519:string)
            n2172 = String To Path(string=w2475) -> (path=w2606:path)
            n2173 = String To Path(string=w2519) -> (path=w2617:path)
            n2174 = local read "Numeric 12"() -> (w2603:i32)
            n2175 = local read "Numeric 8"() -> (w2605:i32)
            n2176 = local read "string1 2"() -> (w2520:string)
            n2177 = local read "string1 4"() -> (w2518:string)
            n2178 = Open/Create/Replace File "Open File"(file path (use dialog)=w2606) -> (refnum out=w2620:refnum<file>, error out=w2619:errorcluster)  [unwired: 5 in, 1 out]
            n2179 = Open/Create/Replace File "Open File"(file path (use dialog)=w2617) -> (refnum out=w2613:refnum<file>, error out=w2614:errorcluster)  [unwired: 5 in, 1 out]
            n2180 = for {
              N: w2605 -> [_]
              tunnel: w2620 -> [w2768]
              tunnel: w2619 -> [w2767]
              tunnel: [w2757] -> w2532 mode=indexing
              tunnel: [w2755] -> w2589 mode=indexing
              tunnel: [w2756] -> w2584 mode=indexing
              tunnel: w2601 -> [_]
              tunnel: [w2749] -> w2586 mode=indexing
              tunnel: [w2745] -> w2555 mode=indexing
              tunnel: [w2741] -> w2530 mode=indexing
              tunnel: [w2737] -> w2511 mode=indexing
              tunnel: [w2732] -> w2471 mode=indexing
              (unwired) TRUE ("line mode (F)")
              # "freq"
              # "Stroke"
              # "Time"
              # "CoF"
              # "Humidity"
              # "Temp"
              # "Air Temp"
              # "ECR"
              n2181 = Read from Text File "Read File"(file (use dialog)=w2768, error in=w2767) -> (text=w2733:string)  [unwired: 2 in, 3 out]
              n2182 = local write "String 6"(w2733) -> ()
              n2183 = String Subset(string=w2733, offset (0)=0, length (rest)=14 ("length (rest)")) -> (substring=w2761:string)
              n2184 = String Subset(string=w2733, offset (0)=35, length (rest)=9 ("length (rest)")) -> (substring=w2758:string)
              n2185 = String Subset(string=w2733, offset (0)=15, length (rest)=9 ("length (rest)")) -> (substring=w2764:string)
              n2186 = Fract/Exp String To Number(string=w2761) -> (number=w2757:dbl)  [unwired: 3 in, 1 out]
              n2187 = Fract/Exp String To Number(string=w2758) -> (number=w2756:dbl)  [unwired: 3 in, 1 out]
              n2188 = Fract/Exp String To Number(string=w2764) -> (number=w2755:dbl)  [unwired: 3 in, 1 out]
              n2189 = String Subset(string=w2733, offset (0)=85, length (rest)=9 ("length (rest)")) -> (substring=w2734:string)
              n2190 = String Subset(string=w2733, offset (0)=25, length (rest)=9 ("length (rest)")) -> (substring=w2740:string)
              n2191 = String Subset(string=w2733, offset (0)=55, length (rest)=9 ("length (rest)")) -> (substring=w2742:string)
              n2192 = String Subset(string=w2733, offset (0)=45, length (rest)=9 ("length (rest)")) -> (substring=w2748:string)
              n2193 = String Subset(string=w2733, offset (0)=65, length (rest)=9 ("length (rest)")) -> (substring=w2754:string)
              n2194 = Fract/Exp String To Number(string=w2740) -> (number=w2737:dbl)  [unwired: 3 in, 1 out]
              n2195 = Fract/Exp String To Number(string=w2734) -> (number=w2732:dbl)  [unwired: 3 in, 1 out]
              n2196 = Fract/Exp String To Number(string=w2742) -> (number=w2741:dbl)  [unwired: 3 in, 1 out]
              n2197 = Fract/Exp String To Number(string=w2748) -> (number=w2745:dbl)  [unwired: 3 in, 1 out]
              n2198 = Fract/Exp String To Number(string=w2754) -> (number=w2751:dbl)  [unwired: 3 in, 1 out]
              n2199 = Add(x=w2751, y=0.0) -> (x+y=w2749:dbl)
            }
            n2200 = for {
              N: w2603 -> [_]
              tunnel: w2614 -> [w2694]
              tunnel: w2613 -> [w2693]
              tunnel: [w2683] -> w2572 mode=indexing
              tunnel: [w2681] -> w2570 mode=indexing
              tunnel: [w2682] -> w2566 mode=indexing
              tunnel: w2601 -> [_]
              tunnel: [w2675] -> w2568 mode=indexing
              tunnel: [w2671] -> w2550 mode=indexing
              tunnel: [w2667] -> w2526 mode=indexing
              tunnel: [w2664] -> w2507 mode=indexing
              tunnel: [w2660] -> w2466 mode=indexing
              (unwired) 9 ("length (rest)")
              (unwired) 9 ("length (rest)")
              (unwired) TRUE ("line mode (F)")
              n2201 = Read from Text File "Read File"(file (use dialog)=w2693, error in=w2694) -> (text=w2661:string)  [unwired: 2 in, 3 out]
              n2202 = local write "String 8"(w2661) -> ()
              n2203 = String Subset(string=w2661, offset (0)=85) -> (substring=w2663:string)  [unwired: 1 in]
              n2204 = String Subset(string=w2661, offset (0)=35, length (rest)=9 ("length (rest)")) -> (substring=w2684:string)
              n2205 = String Subset(string=w2661, offset (0)=55, length (rest)=9 ("length (rest)")) -> (substring=w2669:string)
              n2206 = String Subset(string=w2661, offset (0)=25) -> (substring=w2665:string)  [unwired: 1 in]
              n2207 = String Subset(string=w2661, offset (0)=15, length (rest)=9 ("length (rest)")) -> (substring=w2690:string)
              n2208 = String Subset(string=w2661, offset (0)=0, length (rest)=14 ("length (rest)")) -> (substring=w2687:string)
              n2209 = String Subset(string=w2661, offset (0)=45, length (rest)=9 ("length (rest)")) -> (substring=w2674:string)
              n2210 = String Subset(string=w2661, offset (0)=65, length (rest)=9 ("length (rest)")) -> (substring=w2680:string)
              n2211 = Fract/Exp String To Number(string=w2663) -> (number=w2660:dbl)  [unwired: 3 in, 1 out]
              n2212 = Fract/Exp String To Number(string=w2684) -> (number=w2682:dbl)  [unwired: 3 in, 1 out]
              n2213 = Fract/Exp String To Number(string=w2669) -> (number=w2667:dbl)  [unwired: 3 in, 1 out]
              n2214 = Fract/Exp String To Number(string=w2665) -> (number=w2664:dbl)  [unwired: 3 in, 1 out]
              n2215 = Fract/Exp String To Number(string=w2690) -> (number=w2681:dbl)  [unwired: 3 in, 1 out]
              n2216 = Fract/Exp String To Number(string=w2687) -> (number=w2683:dbl)  [unwired: 3 in, 1 out]
              n2217 = Fract/Exp String To Number(string=w2674) -> (number=w2671:dbl)  [unwired: 3 in, 1 out]
              n2218 = Fract/Exp String To Number(string=w2680) -> (number=w2677:dbl)  [unwired: 3 in, 1 out]
              n2219 = Add(x=w2677, y=0.0) -> (x+y=w2675:dbl)
            }
            n2220 = String To Path(string=w2520) -> (path=w2618:path)
            n2221 = String To Path(string=w2518) -> (path=w2612:path)
            n2222 = local read "Numeric 11"() -> (w2602:i32)
            n2223 = local read "Numeric 13"() -> (w2604:i32)
            n2224 = Open/Create/Replace File "Open File"(file path (use dialog)=w2618) -> (refnum out=w2616:refnum<file>, error out=w2615:errorcluster)  [unwired: 5 in, 1 out]
            n2225 = Open/Create/Replace File "Open File"(file path (use dialog)=w2612) -> (refnum out=w2611:refnum<file>, error out=w2610:errorcluster)  [unwired: 5 in, 1 out]
            n2226 = for {
              N: w2602 -> [_]
              tunnel: w2616 -> [w2731]
              tunnel: w2615 -> [w2730]
              tunnel: [w2720] -> w2582 mode=indexing
              tunnel: [w2718] -> w2580 mode=indexing
              tunnel: [w2719] -> w2575 mode=indexing
              tunnel: w2601 -> [_]
              tunnel: [w2712] -> w2577 mode=indexing
              tunnel: [w2708] -> w2553 mode=indexing
              tunnel: [w2704] -> w2528 mode=indexing
              tunnel: [w2700] -> w2509 mode=indexing
              tunnel: [w2695] -> w2467 mode=indexing
              (unwired) TRUE ("line mode (F)")
              n2227 = Read from Text File "Read File"(file (use dialog)=w2731, error in=w2730) -> (text=w2696:string)  [unwired: 2 in, 3 out]
              n2228 = local write "String 7"(w2696) -> ()
              n2229 = String Subset(string=w2696, offset (0)=85, length (rest)=9 ("length (rest)")) -> (substring=w2699:string)
              n2230 = String Subset(string=w2696, offset (0)=35, length (rest)=9 ("length (rest)")) -> (substring=w2721:string)
              n2231 = String Subset(string=w2696, offset (0)=55, length (rest)=9 ("length (rest)")) -> (substring=w2707:string)
              n2232 = String Subset(string=w2696, offset (0)=25, length (rest)=9 ("length (rest)")) -> (substring=w2701:string)
              n2233 = String Subset(string=w2696, offset (0)=45, length (rest)=9 ("length (rest)")) -> (substring=w2709:string)
              n2234 = String Subset(string=w2696, offset (0)=0, length (rest)=14 ("length (rest)")) -> (substring=w2724:string)
              n2235 = String Subset(string=w2696, offset (0)=15, length (rest)=9 ("length (rest)")) -> (substring=w2727:string)
              n2236 = String Subset(string=w2696, offset (0)=65, length (rest)=9 ("length (rest)")) -> (substring=w2713:string)
              n2237 = Fract/Exp String To Number(string=w2699) -> (number=w2695:dbl)  [unwired: 3 in, 1 out]
              n2238 = Fract/Exp String To Number(string=w2721) -> (number=w2719:dbl)  [unwired: 3 in, 1 out]
              n2239 = Fract/Exp String To Number(string=w2707) -> (number=w2704:dbl)  [unwired: 3 in, 1 out]
              n2240 = Fract/Exp String To Number(string=w2701) -> (number=w2700:dbl)  [unwired: 3 in, 1 out]
              n2241 = Fract/Exp String To Number(string=w2709) -> (number=w2708:dbl)  [unwired: 3 in, 1 out]
              n2242 = Fract/Exp String To Number(string=w2724) -> (number=w2720:dbl)  [unwired: 3 in, 1 out]
              n2243 = Fract/Exp String To Number(string=w2727) -> (number=w2718:dbl)  [unwired: 3 in, 1 out]
              n2244 = Fract/Exp String To Number(string=w2713) -> (number=w2716:dbl)  [unwired: 3 in, 1 out]
              n2245 = Add(x=w2716, y=0.0) -> (x+y=w2712:dbl)
            }
            n2246 = for {
              N: w2604 -> [_]
              tunnel: w2611 -> [w2659]
              tunnel: w2610 -> [w2658]
              tunnel: [w2648] -> w2564 mode=indexing
              tunnel: [w2647] -> w2557 mode=indexing
              tunnel: w2601 -> [_]
              tunnel: [w2636] -> w2562 mode=indexing
              tunnel: [w2641] -> w2559 mode=indexing
              tunnel: [w2637] -> w2549 mode=indexing
              tunnel: [w2632] -> w2524 mode=indexing
              tunnel: [w2628] -> w2505 mode=indexing
              tunnel: [w2623] -> w2465 mode=indexing
              (unwired) 1.0 ("x")
              (unwired) TRUE ("line mode (F)")
              n2247 = Read from Text File "Read File"(file (use dialog)=w2659, error in=w2658) -> (text=w2624:string)  [unwired: 2 in, 3 out]
              n2248 = local write "String 12"(w2624) -> ()
              n2249 = String Subset(string=w2624, offset (0)=85, length (rest)=9 ("length (rest)")) -> (substring=w2626:string)
              n2250 = String Subset(string=w2624, offset (0)=35, length (rest)=9 ("length (rest)")) -> (substring=w2649:string)
              n2251 = String Subset(string=w2624, offset (0)=55, length (rest)=9 ("length (rest)")) -> (substring=w2634:string)
              n2252 = String Subset(string=w2624, offset (0)=25, length (rest)=9 ("length (rest)")) -> (substring=w2630:string)
              n2253 = String Subset(string=w2624, offset (0)=45, length (rest)=9 ("length (rest)")) -> (substring=w2639:string)
              n2254 = String Subset(string=w2624, offset (0)=15, length (rest)=9 ("length (rest)")) -> (substring=w2655:string)
              n2255 = String Subset(string=w2624, offset (0)=0, length (rest)=14 ("length (rest)")) -> (substring=w2652:string)
              n2256 = String Subset(string=w2624, offset (0)=65, length (rest)=9 ("length (rest)")) -> (substring=w2642:string)
              n2257 = Fract/Exp String To Number(string=w2626) -> (number=w2623:dbl)  [unwired: 3 in, 1 out]
              n2258 = Fract/Exp String To Number(string=w2649) -> (number=w2647:dbl)  [unwired: 3 in, 1 out]
              n2259 = Fract/Exp String To Number(string=w2634) -> (number=w2632:dbl)  [unwired: 3 in, 1 out]
              n2260 = Fract/Exp String To Number(string=w2630) -> (number=w2628:dbl)  [unwired: 3 in, 1 out]
              n2261 = Fract/Exp String To Number(string=w2639) -> (number=w2637:dbl)  [unwired: 3 in, 1 out]
              n2262 = Fract/Exp String To Number(string=w2655) -> (number=w2636:dbl)  [unwired: 3 in, 1 out]